vi "ScanDelay_FTIR_BBnorm.vi"() -> ()   [LabVIEW 2022 SP3]
uses:
  Control_scanDelayWorkflow.ctl
  C:/Users/mnopl/OneDrive/Desktop/Software/mnOP.Suite/PRISM/Thorlabs.MotionControl.Controls.dll
  Thorlabs.MotionControl.Controls.dll
  Control_GetSpectrum_BBnorm.ctl
  C:/Users/mnopl/OneDrive/Desktop/Software/mnOP.Suite/PRISM/Thorlabs.MotionControl.FilterFlipperCLI.dll
  Thorlabs.MotionControl.FilterFlipperCLI.dll
panel:
  in  "BB-reference spectrum":bool
  in  "Acquire only\nBB 100% curve with spoofed flip":bool
  in  "Acquire only\nBB 100% curve":bool
  in  "Toggle pause (ms)":dbl=500.0
  out "BB-referenced spectrum (phase)":T1(graph)
  out "BB-referenced spectrum (amplitude)":T1(graph)
  out "Reference BB spectra":dbl[][](array[numeric])
  out "Reference spectra":dbl[][](array[numeric])
  out "Latest replication cmd":string
  in  "Replicate alpha\non accumulation":bool
  out "# Accumulated":i32=2
  in  "Accumulate to #":i32=2
  in  "Cancel\nacquisition":bool
  out "Toggle position":i32=2
  in  "SerialNumber Flipper":string="37005305"
  in  "FilterFlipperControl":refnum<k24>(container)
  out "Spectrum stored":bool=TRUE
  out "Reference stored":bool
  out "Normalized spectrum (phase)":T1(graph)={"Output spectrum"=[1097.4660822342498, 1098.1485860167338, 1098.8310897992178, 1099.5135935817018, 1100.1960973641858, 1100.8786011466698, 1101.5611049291538, 1102.2436087116378, 1102.9261124941218, 1103.6086162766057, 1104.2911200590897, 1104.9736238415737, 1105.6561276240577, 1106.3386314065417, 1107.0211351890257, 1107.7036389715097, 1108.3861427539937, 1109.0686465364777, 1109.7511503189617, 1110.4336541014457, 1111.1161578839296, 1111.7986616664136, 1112.4811654488976, 1113.1636692313816, 1113.8461730138656, 1114.5286767963496, 1115.2111805788336, 1115.8936843613176, 1116.5761881438016, 1117.2586919262856, 1117.9411957087696, 1118.6236994912535, 1119.3062032737375, 1119.9887070562215, 1120.6712108387055, 1121.3537146211895, 1122.0362184036733, 1122.7187221861573, 1123.4012259686413, 1124.0837297511252, 1124.7662335336092, 1125.4487373160932, 1126.1312410985772, 1126.8137448810612, 1127.4962486635452, 1128.1787524460292, 1128.8612562285132, 1129.5437600109972, 1130.2262637934812, 1130.9087675759652, 1131.5912713584491, 1132.2737751409331, 1132.9562789234171, 1133.6387827059011, 1134.321286488385, 1135.003790270869, 1135.686294053353, 1136.368797835837, 1137.051301618321, 1137.733805400805, 1138.416309183289, 1139.098812965773, 1139.781316748257, 1140.463820530741, 1141.146324313225, 1141.828828095709, 1142.511331878193, 1143.193835660677, 1143.876339443161, 1144.558843225645, 1145.241347008129, 1145.923850790613, 1146.606354573097, 1147.288858355581, 1147.971362138065, 1148.653865920549, 1149.336369703033, 1150.018873485517, 1150.701377268001, 1151.383881050485, 1152.0663848329689, 1152.7488886154529, 1153.4313923979369, 1154.1138961804206, 1154.7963999629046, 1155.4789037453886, 1156.1614075278726, 1156.8439113103566, 1157.5264150928406, 1158.2089188753246, 1158.8914226578086, 1159.5739264402926, 1160.2564302227765, 1160.9389340052605, 1161.6214377877445, 1162.3039415702285, 1162.9864453527125, 1163.6689491351965, 1164.3514529176805, 1165.0339567001645, 1165.7164604826485, 1166.3989642651325, 1167.0814680476165, 1167.7639718301004, 1168.4464756125844, 1169.1289793950684, 1169.8114831775524, 1170.4939869600364, 1171.1764907425204, 1171.8589945250044, 1172.5414983074884, 1173.2240020899724], "Output spectrum"=[0.21288449500532583, 0.21143054484736593, 0.21360205749496874, 0.2120631105890475, 0.20990237118245447, 0.2100550965689195, 0.2095359122295658, 0.2092640078801644, 0.20848248343874307, 0.20650169197246354, 0.2057563539123343, 0.20507684171840504, 0.20521349847359482, 0.20596535604203853, 0.20453617772178698, 0.20539187936984576, 0.20838731188545906, 0.20878850241749158, 0.20967541522829136, 0.2097017151015719, 0.20704119738695548, 0.2076753019169947, 0.20918602284923007, 0.20858857733083566, 0.2098655475303692, 0.20992169103994548, 0.20891857261539706, 0.21064865009240577, 0.21042224011211266, 0.2098322090330313, 0.21233872390632724, 0.21235468469552857, 0.21196074819279012, 0.2138709150185505, 0.21314561310626998, 0.21346377727174629, 0.21583371784146907, 0.21507572640098938, 0.21527232748740865, 0.21615586566704167, 0.2149273838744285, 0.21665427259261566, 0.21809876322794203, 0.21652480094189316, 0.21810541510807377, 0.21942143247096924, 0.21866297285037034, 0.2204224686727249, 0.22055890789019725, 0.2198130206226001, 0.22188625318784466, 0.22130773587008234, 0.22091203758926994, 0.2239994779793015, 0.22396141110106593, 0.22406461605897143, 0.2257267081632027, 0.22436492850329612, 0.22561819850296438, 0.2274108697361409, 0.22528214592236864, 0.22663166227073983, 0.22846288647923532, 0.22679518348761, 0.22864349543374585, 0.2299910169374039, 0.2286808145322833, 0.23064530191165866, 0.23070542288562046, 0.23013116157193075, 0.2335181618407221, 0.23301521731104616, 0.2322996298887658, 0.235657379912953, 0.2344459615228607, 0.23388153377453588, 0.23679625841970323, 0.23580000855232966, 0.2373349421923964, 0.24053040228496134, 0.23836946077630108, 0.2398057234782328, 0.2424468980445304, 0.24006185185994836, 0.24159142202012135, 0.24271696807863619, 0.2406319486190728, 0.24395476280655867, 0.24554351199847912, 0.24397185413612701, 0.24642587560721674, 0.24679052495533702, 0.2469078394763994, 0.25021282180383086, 0.24866407816208497, 0.24828430454747738, 0.2524252501610485, 0.25172245134129084, 0.2530429515029453, 0.2561727382627151, 0.2542255154535846, 0.25921162350964233, 0.2633975761430838, 0.25976666589160613, 0.262907039473984, 0.263916317364001, 0.25970502165123804, 0.26402010920952146, 0.2660057820359038, 0.2646334709556704, 0.2706008743147454, 0.27204509753180106]}
  out "Normalized spectrum (amplitude)":T1(graph)={"Output spectrum"=[1097.4660822342498, 1098.1485860167338, 1098.8310897992178, 1099.5135935817018, 1100.1960973641858, 1100.8786011466698, 1101.5611049291538, 1102.2436087116378, 1102.9261124941218, 1103.6086162766057, 1104.2911200590897, 1104.9736238415737, 1105.6561276240577, 1106.3386314065417, 1107.0211351890257, 1107.7036389715097, 1108.3861427539937, 1109.0686465364777, 1109.7511503189617, 1110.4336541014457, 1111.1161578839296, 1111.7986616664136, 1112.4811654488976, 1113.1636692313816, 1113.8461730138656, 1114.5286767963496, 1115.2111805788336, 1115.8936843613176, 1116.5761881438016, 1117.2586919262856, 1117.9411957087696, 1118.6236994912535, 1119.3062032737375, 1119.9887070562215, 1120.6712108387055, 1121.3537146211895, 1122.0362184036733, 1122.7187221861573, 1123.4012259686413, 1124.0837297511252, 1124.7662335336092, 1125.4487373160932, 1126.1312410985772, 1126.8137448810612, 1127.4962486635452, 1128.1787524460292, 1128.8612562285132, 1129.5437600109972, 1130.2262637934812, 1130.9087675759652, 1131.5912713584491, 1132.2737751409331, 1132.9562789234171, 1133.6387827059011, 1134.321286488385, 1135.003790270869, 1135.686294053353, 1136.368797835837, 1137.051301618321, 1137.733805400805, 1138.416309183289, 1139.098812965773, 1139.781316748257, 1140.463820530741, 1141.146324313225, 1141.828828095709, 1142.511331878193, 1143.193835660677, 1143.876339443161, 1144.558843225645, 1145.241347008129, 1145.923850790613, 1146.606354573097, 1147.288858355581, 1147.971362138065, 1148.653865920549, 1149.336369703033, 1150.018873485517, 1150.701377268001, 1151.383881050485, 1152.0663848329689, 1152.7488886154529, 1153.4313923979369, 1154.1138961804206, 1154.7963999629046, 1155.4789037453886, 1156.1614075278726, 1156.8439113103566, 1157.5264150928406, 1158.2089188753246, 1158.8914226578086, 1159.5739264402926, 1160.2564302227765, 1160.9389340052605, 1161.6214377877445, 1162.3039415702285, 1162.9864453527125, 1163.6689491351965, 1164.3514529176805, 1165.0339567001645, 1165.7164604826485, 1166.3989642651325, 1167.0814680476165, 1167.7639718301004, 1168.4464756125844, 1169.1289793950684, 1169.8114831775524, 1170.4939869600364, 1171.1764907425204, 1171.8589945250044, 1172.5414983074884, 1173.2240020899724], "Output spectrum"=[1.0437600267568925, 1.0445294666866474, 1.0397705702891513, 1.0365588077114691, 1.038556721274761, 1.0408095880644594, 1.0424476563660456, 1.0428692410992673, 1.0417194427916883, 1.042850238713553, 1.0440475425444264, 1.0427092918466037, 1.0431196923967452, 1.0440454663973004, 1.0447473293235532, 1.0479997142842818, 1.04850536408959, 1.0461668814541585, 1.0460467202166475, 1.0457146401754922, 1.0463933044283769, 1.0484955227887234, 1.0474983542237284, 1.0474328151154155, 1.0487768327181366, 1.0474428124982593, 1.0472707832372103, 1.0476113135031702, 1.0460943922695316, 1.0467782979860238, 1.0478745871500637, 1.047156974041137, 1.0481225846191404, 1.0482189579589847, 1.0472291373379954, 1.0485426305039969, 1.048028047672481, 1.0471610872248815, 1.049094303588474, 1.0488638922087012, 1.0484987128297814, 1.0493377849679684, 1.046675338879673, 1.045550071522846, 1.0470971505819335, 1.0460065291111194, 1.0462049951250798, 1.0475164570612525, 1.0467302044690008, 1.0474321249218432, 1.04746029744411, 1.045779081687697, 1.047250501022363, 1.047104285756573, 1.0448093335189763, 1.0462009491288433, 1.0460018748830187, 1.044851836987776, 1.0467836879559955, 1.0457891592997033, 1.0444751688237113, 1.0463273936268906, 1.0453109843144839, 1.0448254762878988, 1.04626810932847, 1.04419727475784, 1.0444969618849895, 1.045988661304193, 1.043390055897035, 1.0436837502942822, 1.044152972865949, 1.041413455500755, 1.0433091860896446, 1.0450890001288757, 1.0430312864232871, 1.0437879705711923, 1.0434958674056332, 1.0421501339074697, 1.044090834227986, 1.0427802782233215, 1.0408337583910547, 1.0431022419861884, 1.0427612848025944, 1.0428568360716524, 1.044483019520751, 1.0416194559806138, 1.0419828382024774, 1.0454305025611683, 1.0434276946438128, 1.041748942634975, 1.041288382159901, 1.0398363576550607, 1.0421077463210857, 1.0420827641172203, 1.0390871473904821, 1.041006965526345, 1.0412052253034303, 1.0389370250017262, 1.0411457006925415, 1.040669491810774, 1.0388976461141242, 1.0415516254591484, 1.0410355746019182, 1.0404718837454558, 1.0405907242639103, 1.036256393658658, 1.0375319528927451, 1.0417903322228759, 1.0383900207238663, 1.0374345434138148, 1.040851795081213, 1.040333813003076]}
  in  "Store as reference":bool
  out "Python alpha rep path":path=path "C:/Users/mnopl/Desktop/Software/python/alpha/rep.py"
  out "Activity status":string="Awaiting command"
  out "Acquisition status":string="Ready to acquire spectrum"
  in  "Save spectrum to path":path
  in  "Load reference":bool
  in  "Load reference from path":path
  in  "Load spectrum from path":path
  in  "Apply spectral\nenvelope":bool
  out "Binned interferogram":cluster{"X":dbl, "Y":dbl}[](graph)
  out "Sample BB Spectra":dbl[][](array[numeric])
  out "Sample Spectra":dbl[][](array[numeric])
  out "Python error: spectrum acquisition":errorcluster
  out "Python scandelay path":path=path "C:/Users/mnopl/Desktop/Software/LabVIEW/ScanDelay/scandelay.py"
  in  "Time per\nacquisition (s)":dbl=2.0
  in  "Sampling rate":dbl=250000.0
  in  "Delay calibration\n          factor":dbl=2.403 format="%_6g"
  in  "Cycles per\ninterferogram":i32=1
  in  "Bins per\ninterferogram":i32=30000
  in  "Subtract\nphase slope\n (2pi * dx)":dbl
  out "Python error: DAQ acquisition":errorcluster
  out "Accumulated spectrum (amplitude)":T2(graph)
  out "Acquisition cycle":dbl[][](graph)
  out "% averaged":dbl=100.0
  in  "Pause\nacquisition":bool
  in  "Halt program":bool
  out "Python error: activity loop":errorcluster
  in  "Load spectrum":bool
  in  "Save spectrum":bool
  in  "Normalize spectrum":bool
  in  "Acquire spectrum":bool
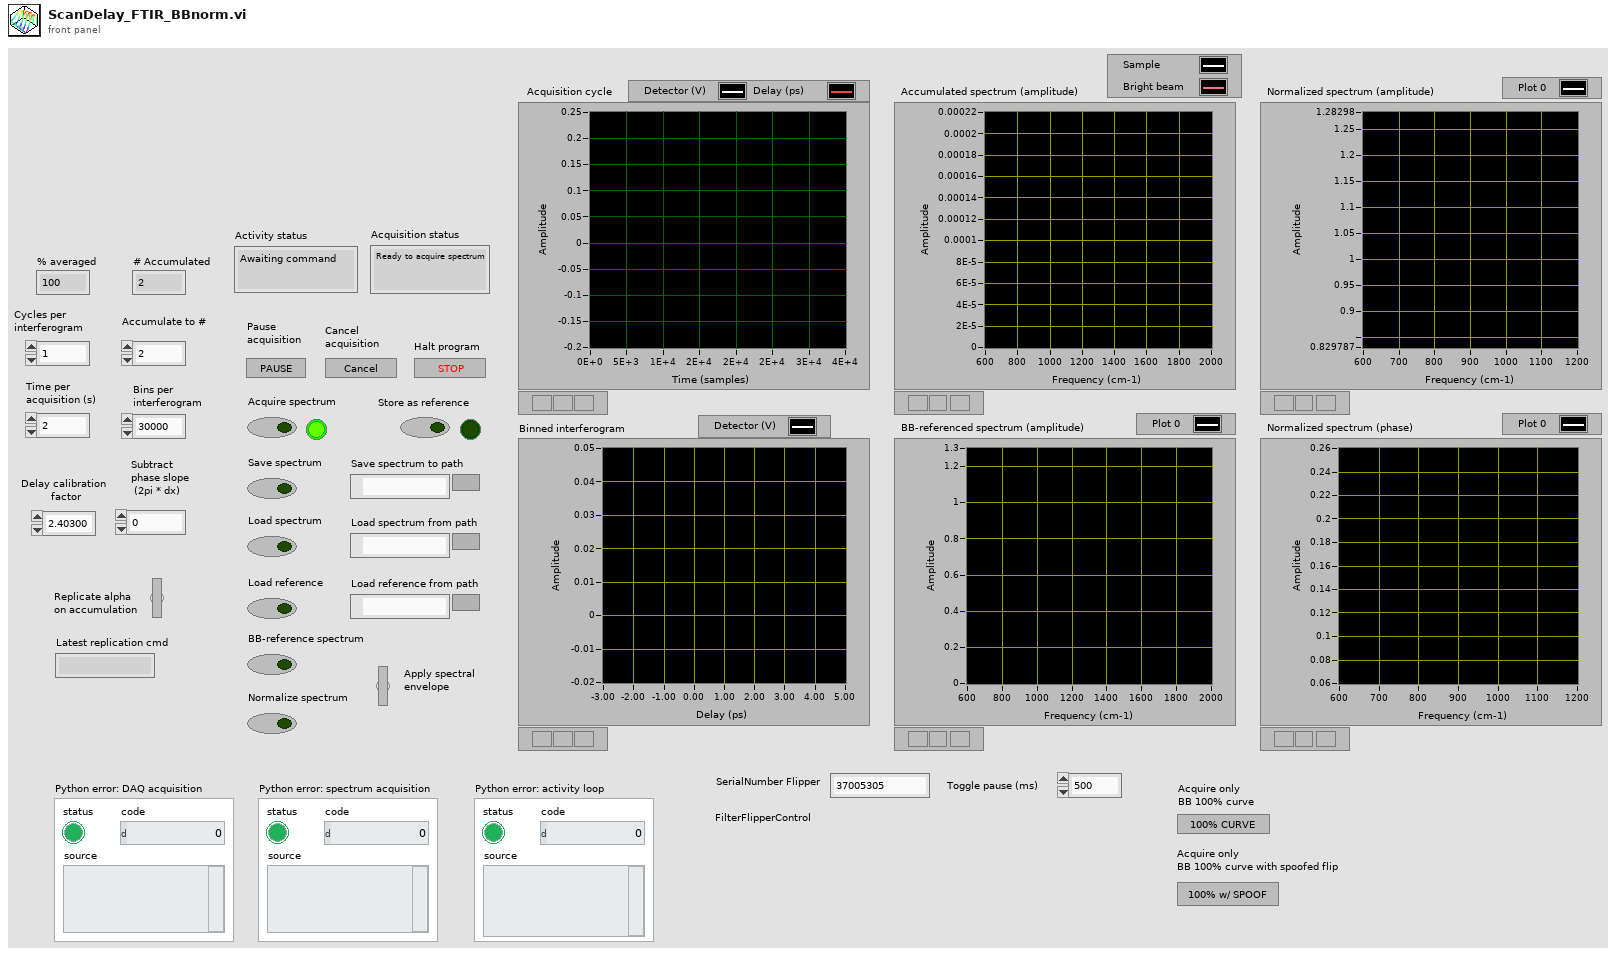
[diagram p1: front panel]
types:
  T1 = cluster{"Output spectrum":dbl[], "Output spectrum":dbl[]}
  T2 = cluster{"Output spectrum":dbl[], "Output spectrum":dbl[]}[]
  T3 = typedef "Control_scanDelayWorkflow.ctl" = enum16{"Initialize", "Sit Idle", "Flip BB", "Load Spectrum", "Store reference", "Save Spectrum", "Load reference", "Check Reference", "Check Spectrum", "BB reference spectrum", "Normalize Spectrum", "Save normalized spectrum", "Done"}
  T4 = typedef "Control_scanDelayWorkflow.ctl" = enum16{"Initialize", "Sit Idle", "BB-reference spectrum", "Load Spectrum", "Store reference", "Save Spectrum", "Load reference", "Check Reference", "Check Spectrum", "Normalize Spectrum", "Done"}
  T5 = cluster{"Sample Spectra":dbl[], "Sample Spectra":dbl[]}
  T6 = typedef "Control_GetSpectrum_BBnorm.ctl" = enum16{"Initialize", "Replicate alpha", "Flip in BB", "Get Spectrum", "Accumulate BB spectrum", "Flip out BB", "Accumulate sample spectrum", "Assess accumulation", "Finalize", "Done"}
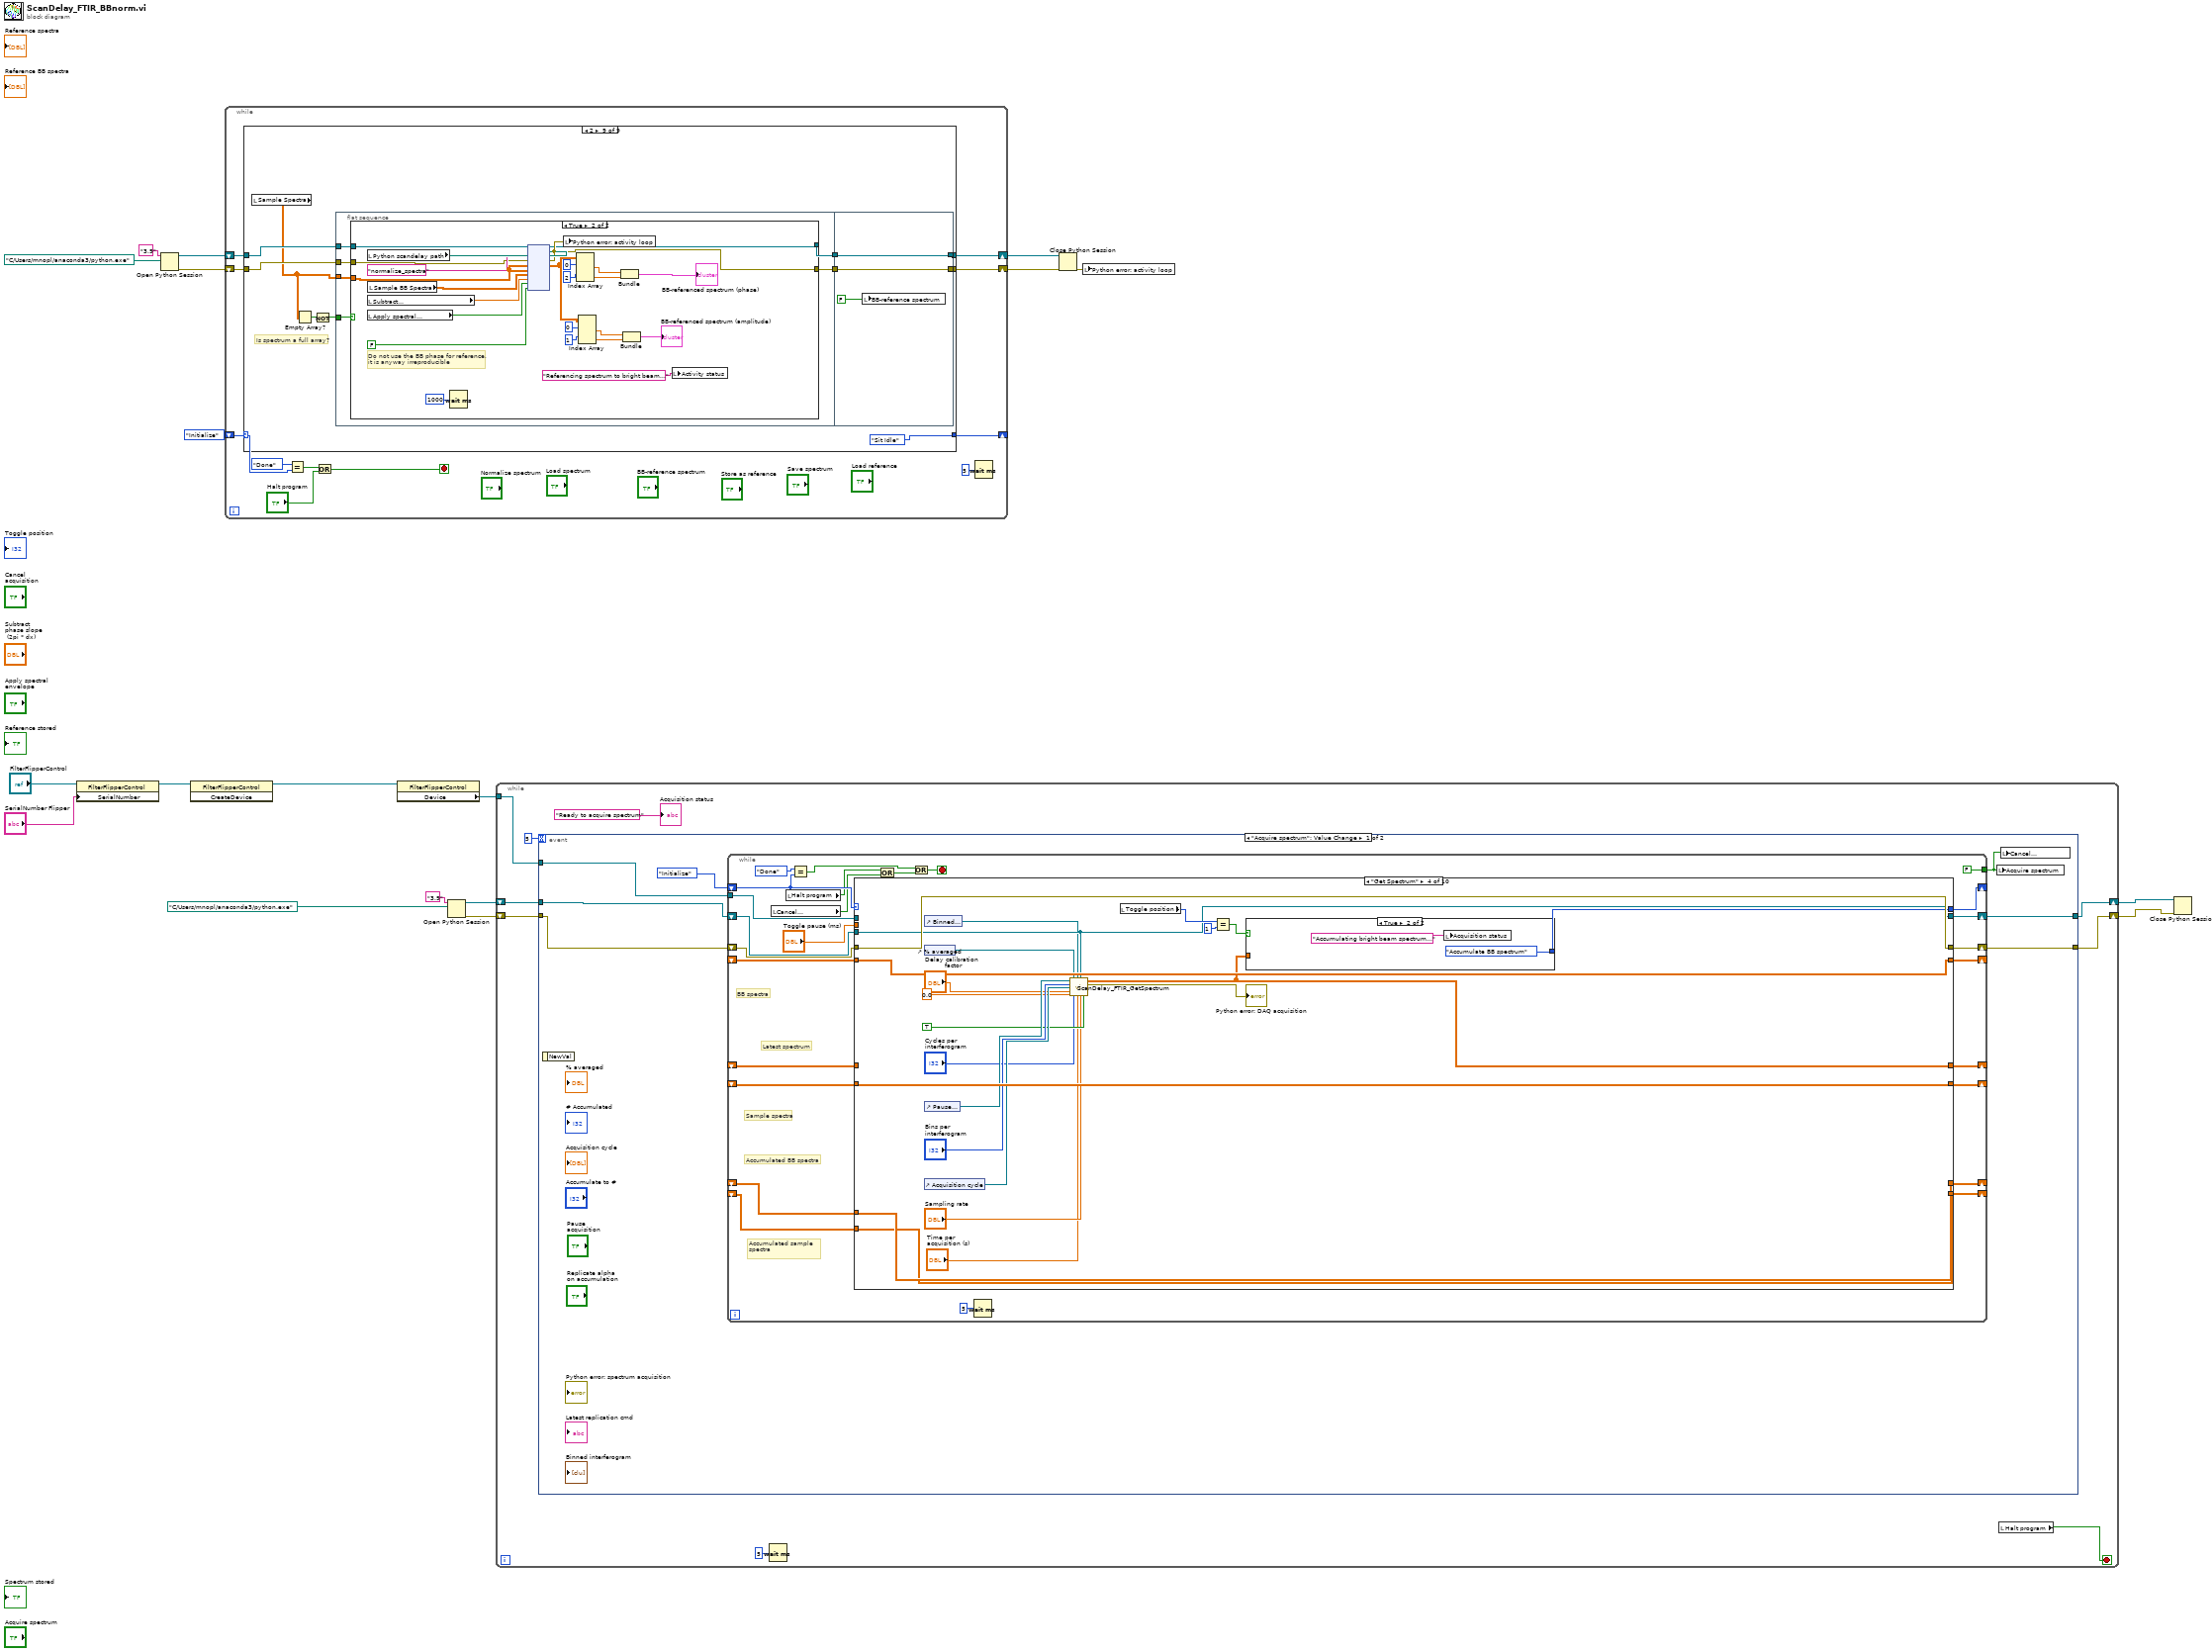
[diagram p0: block diagram]
diagram:
  n1 = property class="FilterFlipperControl"(reference="FilterFlipperControl", "SerialNumber"="SerialNumber Flipper") -> (reference out=w10:refnum<k24>)  [unwired: 1 in, 1 out]
  n2 = Open Python Session(python version="3.9", python path=path "C:/Users/mnopl/anaconda3/python.exe") -> (session out=w15:refnum<k35>, error out=w14:errorcluster)  [unwired: 1 in]
  n3 = invoke class="FilterFlipperControl" method="CreateDevice"(reference=w10) -> (reference out=w9:refnum<k24>)  [unwired: 2 in, 2 out]
  n4 = while {
    shift-right: [w22] -> _
    shift-left: Control_scanDelayWorkflow."Initialize" -> [w28]
    shift-right: [w29] -> w16
    shift-left: w14 -> [w20]
    shift-right: [w23] -> w17
    shift-left: w15 -> [w21]
    stop <- w26 stop-if-true
    n5 = case shown="2" w28 {
      selector: w28 -> [_ _ _ _ _ w121 _ _ _]
      tunnel: [w34 w60 w70 w72 w79 w122 w125 w132 w144] -> w29
      tunnel: w21 -> [w35 w59 w69 w73 w82 w123 w126 w133 w142]
      tunnel: w20 -> [w34 w60 w70 w72 w81 w122 w125 w132 w141]
      tunnel: [w35 w59 w69 w73 w80 w123 w126 w133 w143] -> w23
      tunnel: [w33 Control_scanDelayWorkflow."Sit Idle" Control_scanDelayWorkflow."Sit Idle" Control_scanDelayWorkflow."Sit Idle" Control_scanDelayWorkflow."Sit Idle" w121 Control_scanDelayWorkflow."Sit Idle" Control_scanDelayWorkflow."Sit Idle" Control_scanDelayWorkflow."Sit Idle"] -> w22
      frame 1, Default {
        n6 = event shown="[0] \"Normalize spectrum\": Value Change" {
          selector: _ -> [_ _ _ _ _]
          dyn-events: _ -> [_ _ _ _ _]
          timeout: 5 -> [_ _ _ _ w52]
          tunnel: [w36 w40 w47 w48 Control_scanDelayWorkflow."Sit Idle"] -> w33
          event "Normalize spectrum": Value Change {
            n7 = event-data() -> ("NewVal"=w37:bool)  [unwired: 1 in]
            n8 = Select(t=Control_scanDelayWorkflow."Normalize Spectrum", s=w37, f=Control_scanDelayWorkflow."Sit Idle") -> (s? t:f=w36:T3)
          }
          event "Store as reference": Value Change {
            n9 = event-data() -> ("NewVal"=w43:bool)  [unwired: 1 in]
            n10 = Select(t=Control_scanDelayWorkflow."Store reference", s=w43, f=Control_scanDelayWorkflow."Sit Idle") -> (s? t:f=w40:T3)
          }
          event "BB-reference spectrum": Value Change {
            n11 = event-data() -> ("NewVal"=w45:bool)  [unwired: 1 in]
            n12 = Select(t=Control_scanDelayWorkflow."BB-reference spectrum", s=w45, f=Control_scanDelayWorkflow."Sit Idle") -> (s? t:f=w47:u16)
          }
          event "Save spectrum": Value Change {
            n13 = event-data() -> ("NewVal"=w49:bool)  [unwired: 1 in]
            n14 = Select(t=Control_scanDelayWorkflow."Save Spectrum", s=w49, f=Control_scanDelayWorkflow."Sit Idle") -> (s? t:f=w48:T3)
          }
          event Timeout {
            n15 = event-data() -> ()  [unwired: 1 in, 2 out]
            n16 = Wait (ms)(milliseconds to wait=w52) -> ()  [unwired: 1 out]
          }
        }
        "Activity status" <- "Awaiting command"
      }
      frame 4 {
        # "Is spectrum a full array?"
        n17 = local read "Sample Spectra"() -> (w55:dbl[][])
        n18 = local read "Sample BB Spectra"() -> (w54:dbl[][])
        n19 = Empty Array?(array=w55) -> (empty?=w57:bool)
        n20 = Not(x=w57) -> (.not. x?=w56:bool)
        n21 = case shown="True" w56 {
          tunnel: w55 -> [_ w63]
          tunnel: w54 -> [_ w64]
          frame False {
            n22 = Wait (ms)(milliseconds to wait=1000) -> ()  [unwired: 1 out]
            n23 = local write "Activity status"("Error: Spectrum is empty!") -> ()
          }
          frame True {
            n24 = local write "Reference BB spectra"(w64) -> ()
            n25 = local write "Reference spectra"(w63) -> ()
            n26 = local write "Reference stored"(TRUE) -> ()
            n27 = Wait (ms)(milliseconds to wait=1000) -> ()  [unwired: 1 out]
            n28 = local write "Activity status"("Storing reference!") -> ()
          }
        }
      }
      frame 5 {
      }
      frame 6 {
      }
      frame 10 {
        n29 = local read "Reference stored"() -> (w76:bool)
        n30 = local read "Spectrum stored"() -> (w75:bool)
        n31 = And(x=w75, y=w76) -> (x .and. y?=w74:bool)
        n32 = flat-sequence {
          tunnel: w82 -> [w88]
          tunnel: w81 -> [w87]
          tunnel: [w86] -> w78
          tunnel: [w85] -> w77
          tunnel: w74 -> [w84]
          tunnel: [w119] -> w79
          tunnel: [w120] -> w80
          tunnel: w78 -> [w120]
          tunnel: w77 -> [w119]
          frame #0 {
            n33 = case shown="True" w84 {
              tunnel: w88 -> [w90 w116]
              tunnel: w87 -> [w89 w115]
              tunnel: [w90 w114] -> w86
              tunnel: [w89 w97] -> w85
              frame False {
                n34 = Wait (ms)(milliseconds to wait=1000) -> ()  [unwired: 1 out]
                n35 = local write "Activity status"("Error: Spectrum or reference is empty!") -> ()
              }
              frame True {
                n36 = Wait (ms)(milliseconds to wait=1000) -> ()  [unwired: 1 out]
                n37 = local read "Python scandelay path"() -> (w113:path)
                n38 = local read "Sample Spectra"() -> (w98:dbl[][])
                n39 = local read "Sample BB Spectra"() -> (w99:dbl[][])
                n40 = local read "Reference spectra"() -> (w94:dbl[][])
                n41 = local read "Reference BB spectra"() -> (w93:dbl[][])
                n42 = local read "Subtract\nphase slope\n (2pi * dx)"() -> (w95:dbl)
                n43 = local read "Apply spectral\nenvelope"() -> (w96:bool)
                n44 = local write "Activity status"("Normalizing spectrum!") -> ()
                n45 = node(w116, w113, "double_normalize_spectra", w115, w98, w98, w99, w94, w93, w95, w96) -> (w114:refnum<k35>, w97:errorcluster, w101:dbl[][])  [unwired: 6 in, 2 out]
                "Python error: activity loop" <- w97
                n46 = Index Array(array=w101, index (row) #1=0, index (row) #2=1) -> (element #1=w109:dbl[], element #2=w108:dbl[])  [unwired: 2 in]
                n47 = Index Array(array=w101, index (row) #1=0, index (row) #2=2) -> (element #1=w105:dbl[], element #2=w104:dbl[])  [unwired: 2 in]
                n48 = Bundle("Sample Spectra"=w109, "Sample Spectra"=w108) -> (→"Normalized spectrum (amplitude)":T5)  [unwired: 1 in]
                n49 = Bundle("Sample Spectra"=w105, "Sample Spectra"=w104) -> (→"Normalized spectrum (phase)":T5)  [unwired: 1 in]
              }
            }
          }
          frame #1 {
            n50 = local write "Normalize spectrum"(FALSE) -> ()
          }
        }
      }
      frame 12 {
      }
      frame 3 {
      }
      frame 0 {
        n51 = local write "Acquire spectrum"(FALSE) -> ()
        n52 = local write "Reference stored"(FALSE) -> ()
        n53 = local write "Spectrum stored"(FALSE) -> ()
        "Python scandelay path" <- path "C:/Users/mnopl/Desktop/Software/LabVIEW/ScanDelay/scandelay.py"
        "Python alpha rep path" <- path "C:/Users/mnopl/Desktop/Software/python/alpha/rep.py"
      }
      frame 2 {
        # "Is spectrum a full array?"
        n54 = local read "Sample Spectra"() -> (w135:dbl[][])
        n55 = Empty Array?(array=w135) -> (empty?=w137:bool)
        n56 = Not(x=w137) -> (.not. x?=w136:bool)
        n57 = flat-sequence {
          tunnel: w142 -> [w148]
          tunnel: w141 -> [w147]
          tunnel: w136 -> [w146]
          tunnel: [w150] -> w139
          tunnel: [w149] -> w138
          tunnel: w135 -> [w145]
          tunnel: [w180] -> w143
          tunnel: [w181] -> w144
          tunnel: w139 -> [w181]
          tunnel: w138 -> [w180]
          frame #0 {
            n58 = case shown="True" w146 {
              tunnel: [w151 w162] -> w150
              tunnel: [w152 w161] -> w149
              tunnel: w148 -> [w152 w160]
              tunnel: w147 -> [w151 w159]
              tunnel: w145 -> [_ w155]
              frame False {
                n59 = Wait (ms)(milliseconds to wait=1000) -> ()  [unwired: 1 out]
                n60 = local write "Activity status"("Error: Spectrum or reference is empty!") -> ()
              }
              frame True {
                # "Do not use the BB phase for reference,\nit is anyway irreproducible"
                n61 = local read "Python scandelay path"() -> (w172:path)
                n62 = local read "Subtract\nphase slope\n (2pi * dx)"() -> (w171:dbl)
                n63 = local read "Apply spectral\nenvelope"() -> (w170:bool)
                n64 = local read "Sample BB Spectra"() -> (w158:dbl[][])
                n65 = Wait (ms)(milliseconds to wait=1000) -> ()  [unwired: 1 out]
                n66 = node(w160, w172, "normalize_spectra", w159, w155, w155, w158, w171, w170, FALSE) -> (w161:refnum<k35>, w162:errorcluster, w169:dbl[][])  [unwired: 5 in, 2 out]
                n67 = local write "Python error: activity loop"(w162) -> ()
                n68 = Index Array(array=w169, index (row) #1=0, index (row) #2=2) -> (element #1=w175:dbl[], element #2=w174:dbl[])  [unwired: 2 in]
                n69 = Index Array(array=w169, index (row) #1=0, index (row) #2=1) -> (element #1=w178:dbl[], element #2=w177:dbl[])  [unwired: 2 in]
                n70 = Bundle("Sample Spectra"=w175, "Sample Spectra"=w174) -> (→"BB-referenced spectrum (phase)":T5)  [unwired: 1 in]
                n71 = Bundle("Sample Spectra"=w178, "Sample Spectra"=w177) -> (→"BB-referenced spectrum (amplitude)":T5)  [unwired: 1 in]
                n72 = local write "Activity status"("Referencing spectrum to bright beam...") -> ()
              }
            }
          }
          frame #1 {
            n73 = local write "BB-reference spectrum"(FALSE) -> ()
          }
        }
      }
    }
    n74 = Equal?(x=Control_scanDelayWorkflow."Done", y=w28) -> (x = y?=w24:bool)
    n75 = Or(x=w24, y="Halt program") -> (x .or. y?=w26:bool)
    n76 = Wait (ms)(milliseconds to wait=5) -> ()  [unwired: 1 out]
  }
  n77 = property class="FilterFlipperControl"(reference=w9) -> ("Device"=w3:refnum<k24>)  [unwired: 1 in, 2 out]
  n78 = Open Python Session(python version="3.9", python path=path "C:/Users/mnopl/anaconda3/python.exe") -> (session out=w5:refnum<k35>, error out=w4:errorcluster)  [unwired: 1 in]
  n79 = while {
    tunnel: w3 -> [w184]
    shift-right: [w182] -> w1
    shift-left: w4 -> [w185]
    shift-right: [w183] -> w2
    shift-left: w5 -> [w186]
    stop <- w190 stop-if-true
    n80 = event shown="[0] \"Acquire spectrum\": Value Change" {
      selector: _ -> [_ _]
      dyn-events: _ -> [_ _]
      timeout: 5 -> [_ w431]
      tunnel: w186 -> [w196 w430]
      tunnel: w185 -> [w195 w429]
      tunnel: w184 -> [w194 _]
      tunnel: [w193 w430] -> w183
      tunnel: [w192 w429] -> w182
      event "Acquire spectrum": Value Change {
        n81 = event-data() -> ()  [unwired: 1 in, 1 out]
        n82 = while {
          shift-right: [w221] -> _
          shift-left: _ -> [w220]
          shift-right: [w222] -> _
          shift-left: _ -> [w219]
          shift-right: [w218] -> _
          shift-left: Control_GetSpectrum_BBnorm."Initialize" -> [w211]
          shift-right: [w215] -> w192
          shift-left: w195 -> [w216]
          shift-right: [w214] -> w193
          shift-left: w196 -> [w217]
          shift-right: [w213] -> _
          shift-left: _ -> [w205]
          tunnel: w194 -> [w204]
          tunnel: [FALSE] -> w191
          shift-right: [w201] -> _
          shift-left: _ -> [w199]
          shift-right: [w200] -> _
          shift-left: _ -> [w198]
          stop <- w206 stop-if-true
          # "Accumulated BB spectra"
          # "Accumulated sample spectra"
          # "Sample spectra"
          # "Latest spectrum"
          # "BB spectra"
          n83 = local read "Cancel\nacquisition"() -> (w208:bool)
          n84 = local read "Halt program"() -> (w209:bool)
          n85 = Equal?(x=Control_GetSpectrum_BBnorm."Done", y=w211) -> (x = y?=w210:bool)
          n86 = case shown="\"Get Spectrum\"" w211 {
            tunnel: [w224 w250 w257 w289 w301 w341 w365 w387 w414 w424] -> w222
            tunnel: [w224 w251 w258 w288 w316 w342 w358 w388 w413 w426] -> w221
            tunnel: w220 -> [_ w251 w258 w288 w325 w342 w358 w388 w413 w426]
            tunnel: w219 -> [_ w250 w257 w289 w301 w341 w366 w387 w414 w424]
            tunnel: [w231 Control_GetSpectrum_BBnorm."Flip in BB" Control_GetSpectrum_BBnorm."Get Spectrum" w284 w309 Control_GetSpectrum_BBnorm."Get Spectrum" Control_GetSpectrum_BBnorm."Assess accumulation" w392 Control_GetSpectrum_BBnorm."Done" Control_GetSpectrum_BBnorm."Done"] -> w218
            tunnel: w217 -> [w228 w247 w260 w281 w320 w340 w378 w394 w416 w428]
            tunnel: w216 -> [w227 w246 w259 w290 w319 w339 w377 w395 w415 w427]
            tunnel: [w227 w239 w259 w290 w307 w339 w364 w395 w415 w427] -> w215
            tunnel: [w228 w240 w260 w281 w318 w340 w376 w394 w416 w428] -> w214
            tunnel: w204 -> [_ _ w255 _ _ w337 _ _ _ _]
            tunnel: [w224 w238 w256 w269 w310 w338 w369 w391 w420 w425] -> w213
            tunnel: w205 -> [_ w238 w256 _ w310 w338 w369 w391 w420 w425]
            tunnel: "Toggle pause (ms)" -> [_ _ w254 _ _ w336 _ _ _ _]
            tunnel: [w224 w237 w253 w283 w297 w335 w355 w390 w418 w422] -> w201
            tunnel: [w224 w236 w252 w282 w295 w334 w356 w389 w417 w421] -> w200
            tunnel: w199 -> [_ w237 w253 w283 w295 w335 w355 w390 w418 w422]
            tunnel: w198 -> [_ w236 w252 w282 w296 w334 _ w389 w417 w421]
            frame "Initialize", Default {
              w232 = dbl[] []
              n87 = local write "Toggle position"(1) -> ()
              n88 = local write "# Accumulated"(0) -> ()
              n89 = local write "Spectrum stored"(FALSE) -> ()
              n90 = local read "Replicate alpha\non accumulation"() -> (w229:bool)
              n91 = case shown="False" w229 {
                tunnel: [Control_GetSpectrum_BBnorm."Flip in BB" Control_GetSpectrum_BBnorm."Replicate alpha"] -> w231
                frame False {
                }
                frame True {
                  n92 = local write "Acquisition status"("Replicating alpha...") -> ()
                }
              }
              n93 = Build Array(w232, w232) -> (w224:dbl[][])
              "Sample Spectra" <- w224
              "Sample BB Spectra" <- w224
            }
            frame "Replicate alpha" {
              w244 = "replicate"
              # "Wait time for replication (s)"
              n94 = local read "# Accumulated"() -> (w242:i32)
              n95 = local write "Acquisition status"("Replicating alpha...") -> ()
              n96 = local read "Python alpha rep path"() -> (w245:path)
              n97 = node(w247, w245, w244, w246, w244, w242, 8) -> (w240:refnum<k35>, w239:errorcluster, w241:string)  [unwired: 2 in, 2 out]
              n98 = local write "Python error: spectrum acquisition"(w239) -> ()
              n99 = local write "Latest replication cmd"(w241) -> ()
            }
            frame "Flip in BB" {
              n100 = flat-sequence {
                tunnel: w255 -> [w265]
                tunnel: w254 -> [w266]
                frame #0 {
                  n101 = local write "Acquisition status"("Toggling to bright beam...") -> ()
                }
                frame #1 {
                  w264 = 1
                  n102 = local write "Toggle position"(w264) -> ()
                  n103 = invoke class="FilterFlipper" method="SetPosition"(reference=w265, "position"=w264, "waitTimeout"=20000) -> ()  [unwired: 2 in, 5 out]
                }
                frame #2 {
                  n104 = Wait (ms)(milliseconds to wait=w266) -> ()  [unwired: 1 out]
                  n105 = local write "Acquisition status"("Acquiring bright beam spectrum...") -> ()
                }
              }
            }
            frame "Get Spectrum" {
              n106 = control-ref of="Binned interferogram"() -> (w280:refnum<vi>)
              n107 = control-ref of="% averaged"() -> (w279:refnum<vi>)
              n108 = control-ref of="Pause\nacquisition"() -> (w278:refnum<vi>)
              n109 = control-ref of="Acquisition cycle"() -> (w276:refnum<vi>)
              n110 = call "ScanDelay_FTIR_GetSpectrum.vi"("Acquire / Pause? External"=w278, "% averaged (external)"=w279, "Binned interferogram (external)"=w280, "Python refnum in"=w281, "N delays"="Bins per\ninterferogram", "Acquisition cycle (external)"=w276, "Delay calibration\n          factor"="Delay calibration\n          factor", "Subtract\ndelay (ps)"=0.0, "Acquisitions per interferogram"="Cycles per\ninterferogram", "Time per acquisition (s)"="Time per\nacquisition (s)", "Sampling rate"="Sampling rate", "Extract envelope"=TRUE) -> ("Output spectrum"=w269:dbl[][], "Python error out"=→"Python error: DAQ acquisition":errorcluster)  [unwired: 2 in]
              n111 = local read "Toggle position"() -> (w287:i32)
              n112 = Equal?(x=w287, y=1) -> (x = y?=w285:bool)
              n113 = case shown="True" w285 {
                tunnel: [Control_GetSpectrum_BBnorm."Accumulate sample spectrum" Control_GetSpectrum_BBnorm."Accumulate BB spectrum"] -> w284
                tunnel: w269 -> [_ _]
                frame False {
                  n114 = local write "Acquisition status"("Accumulating sample spectrum...") -> ()
                }
                frame True {
                  n115 = local write "Acquisition status"("Accumulating bright beam spectrum...") -> ()
                }
              }
            }
            frame "Accumulate BB spectrum" {
              n116 = local read "# Accumulated"() -> (w324:i32)